vi "SMain.vi"() -> ()   [LabVIEW 2011] (continued)
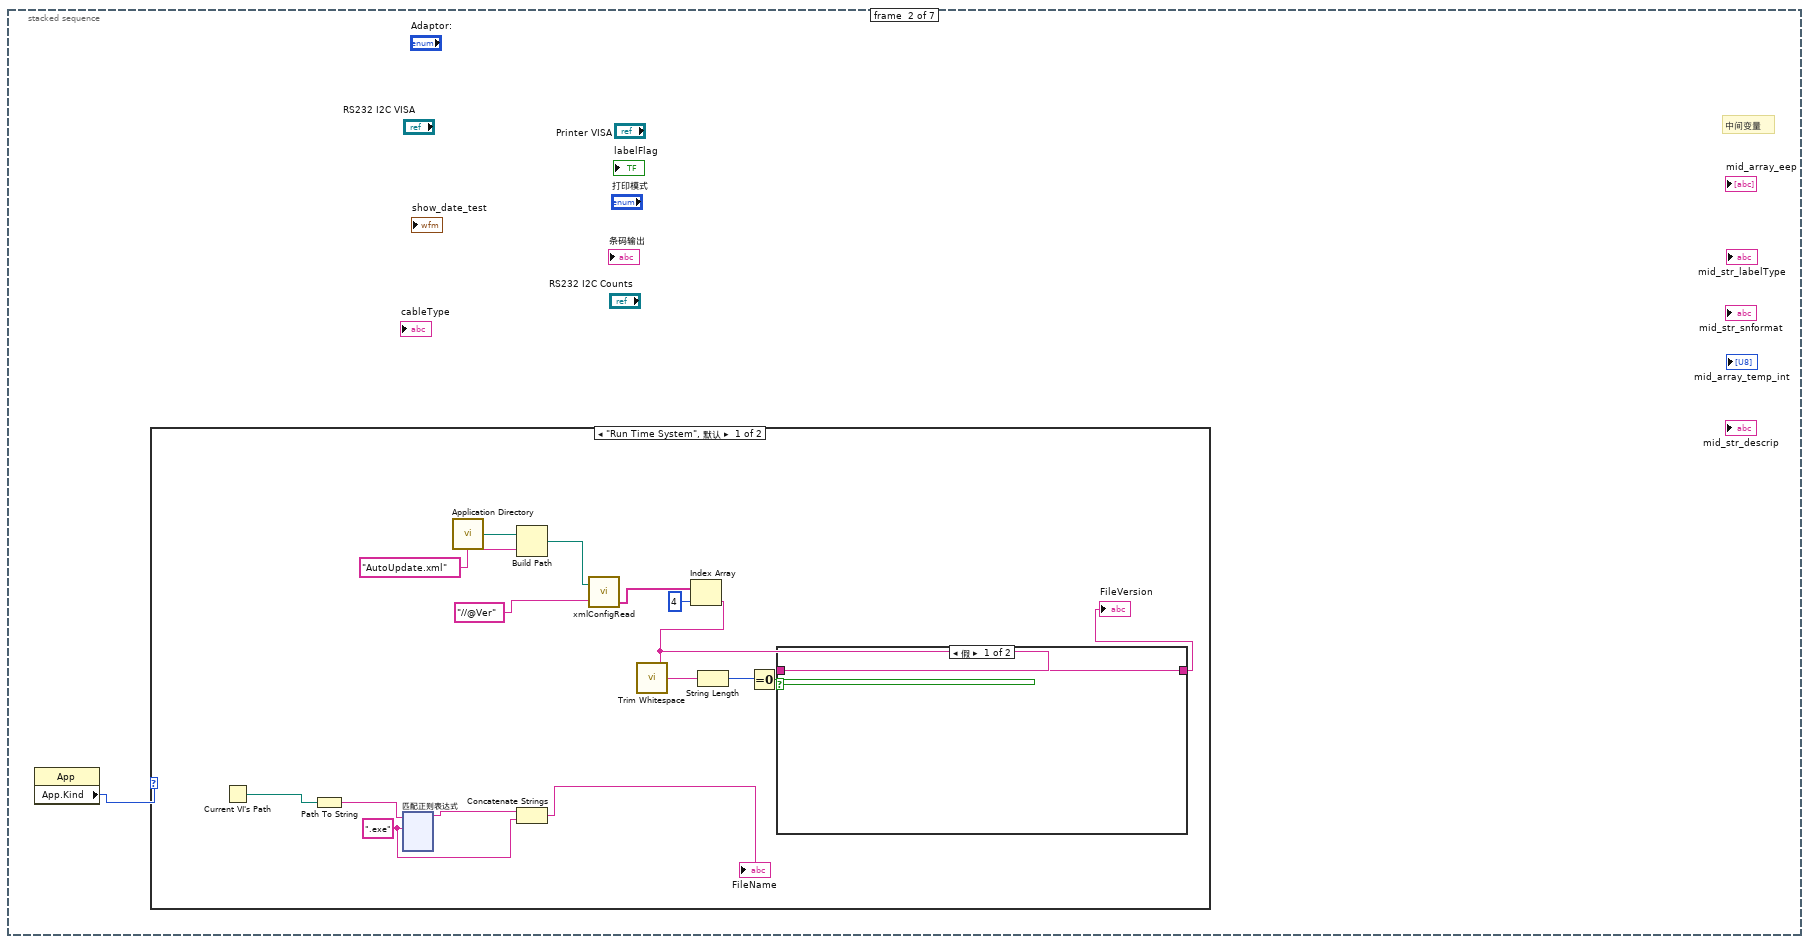
[diagram p4: hidden frame]
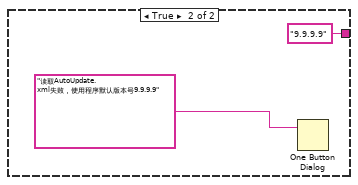
[diagram p5: hidden frame]
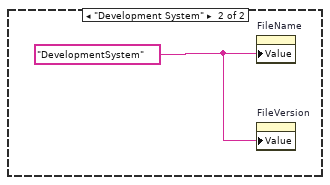
[diagram p6: hidden frame]
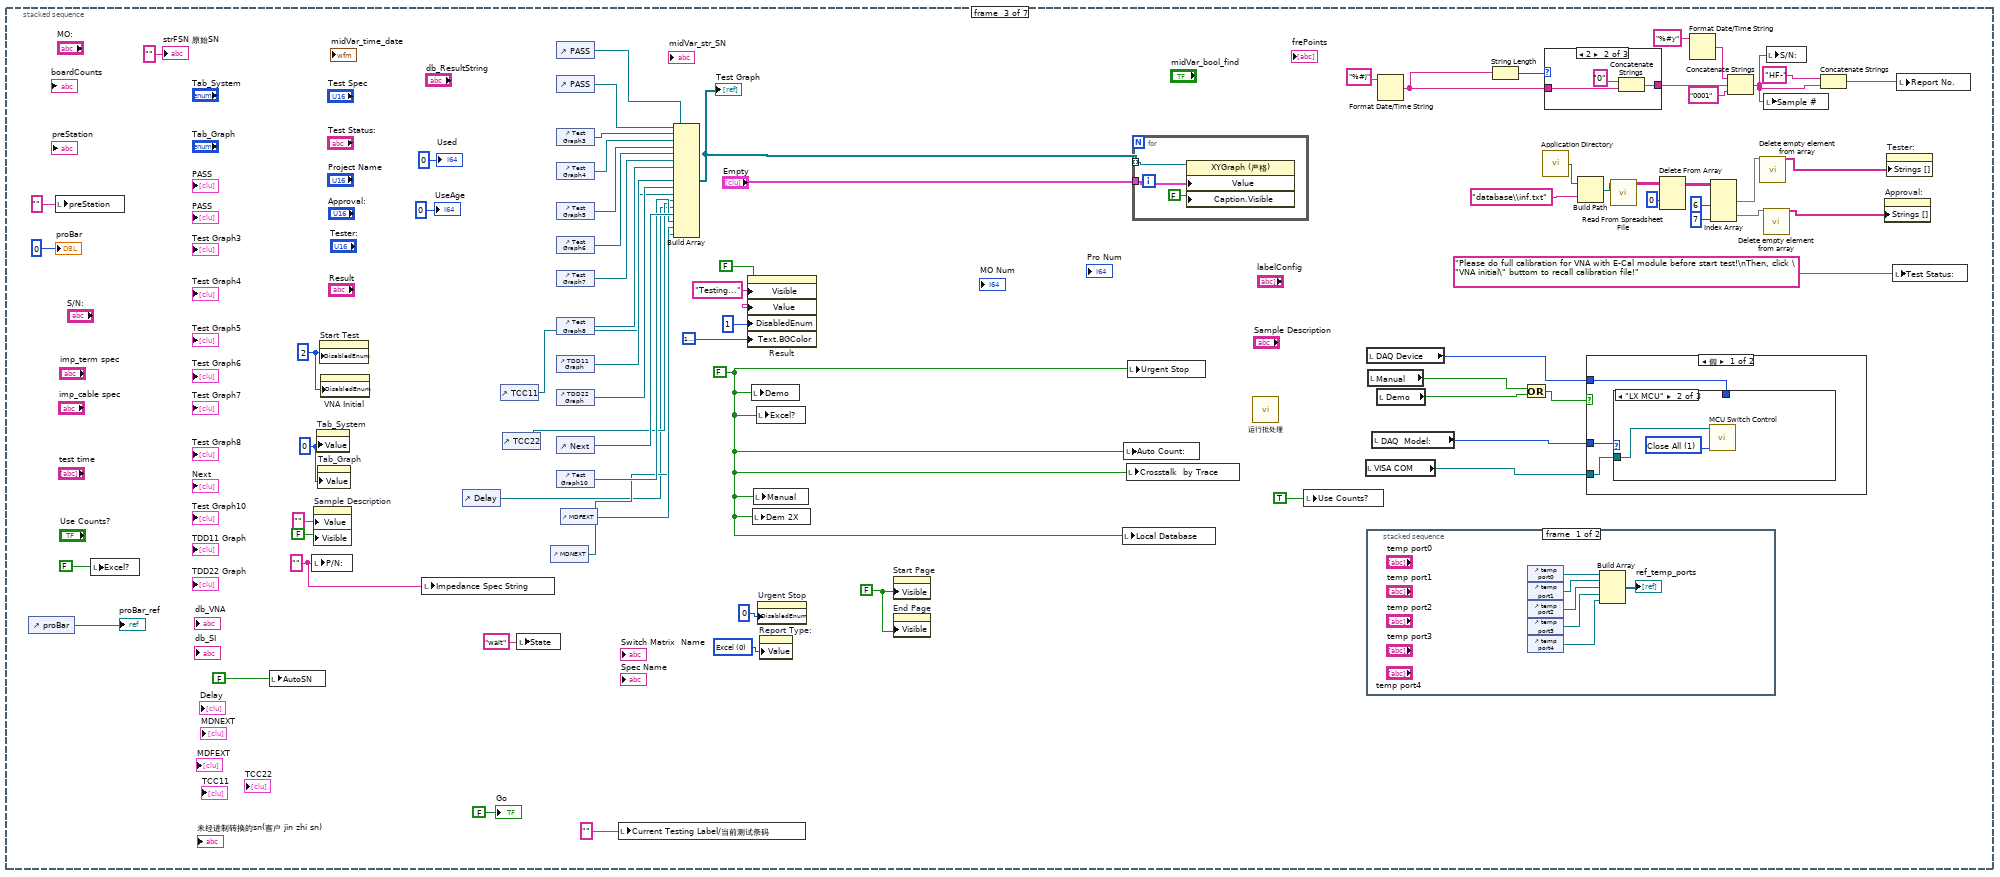
[diagram p7: hidden frame]
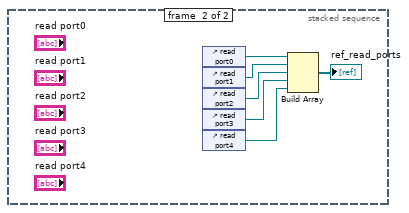
[diagram p8: hidden frame]
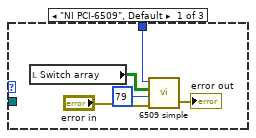
[diagram p9: hidden frame]
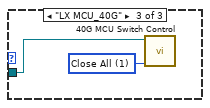
[diagram p10: hidden frame]
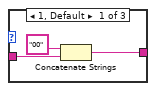
[diagram p12: hidden frame]
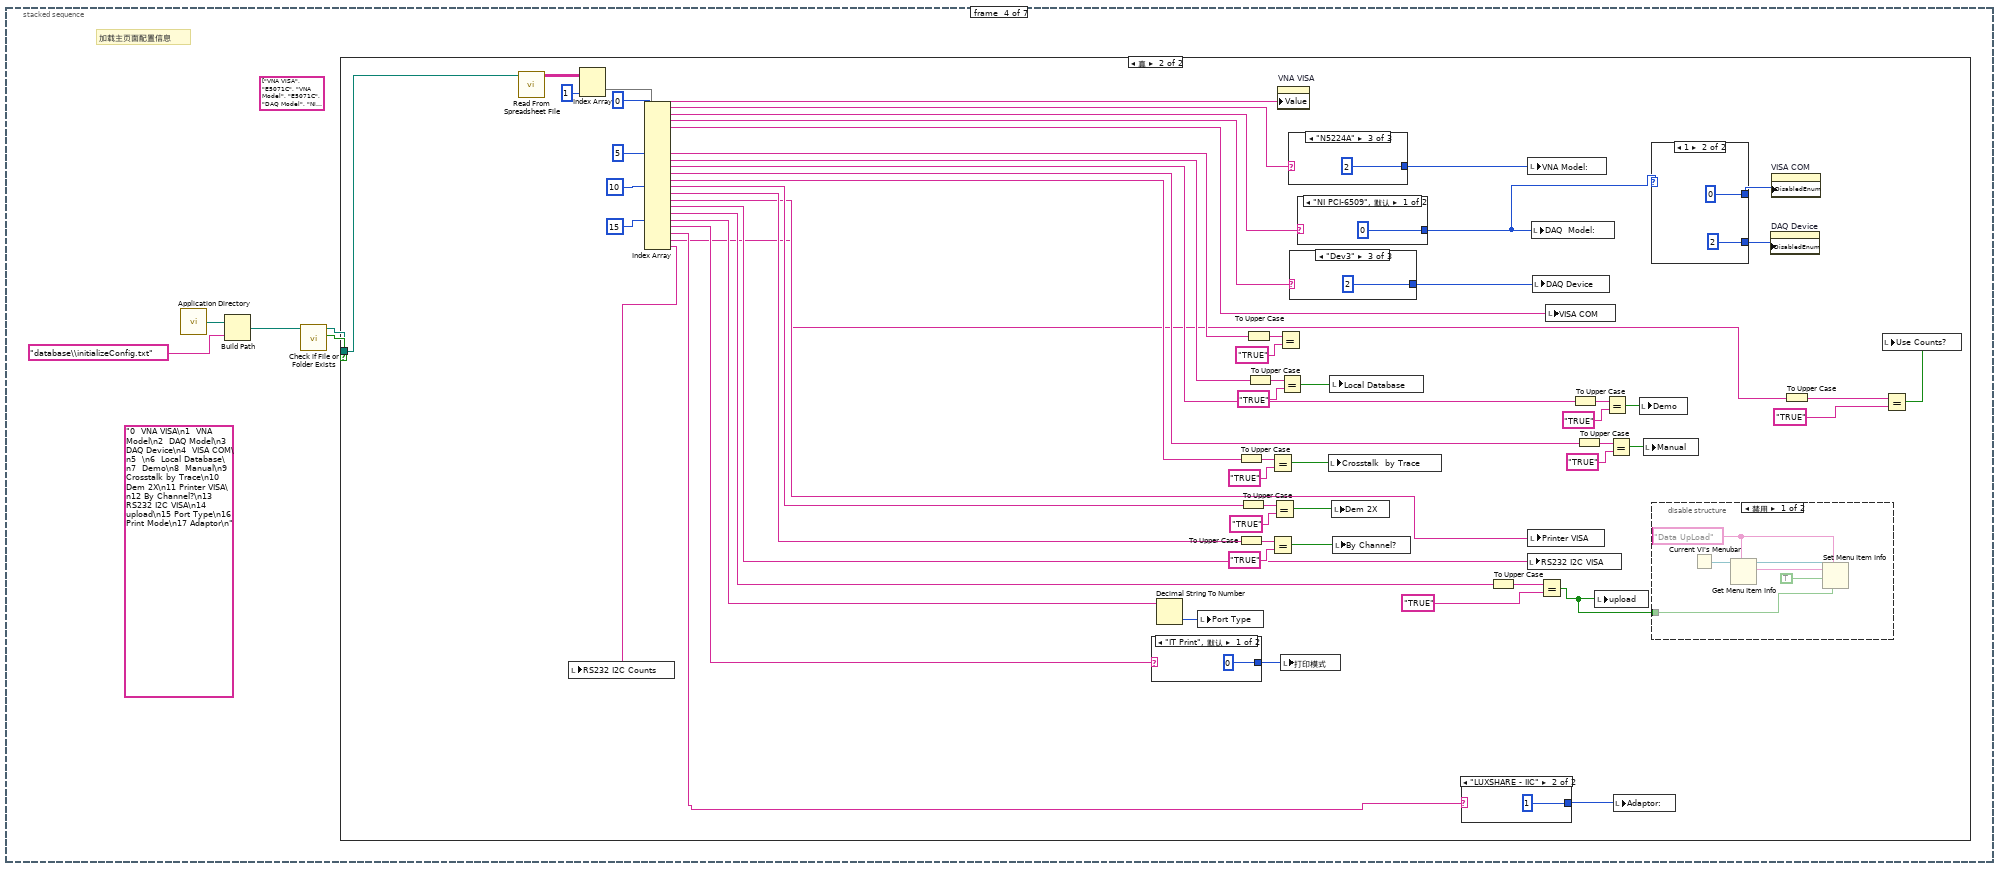
[diagram p14: hidden frame]
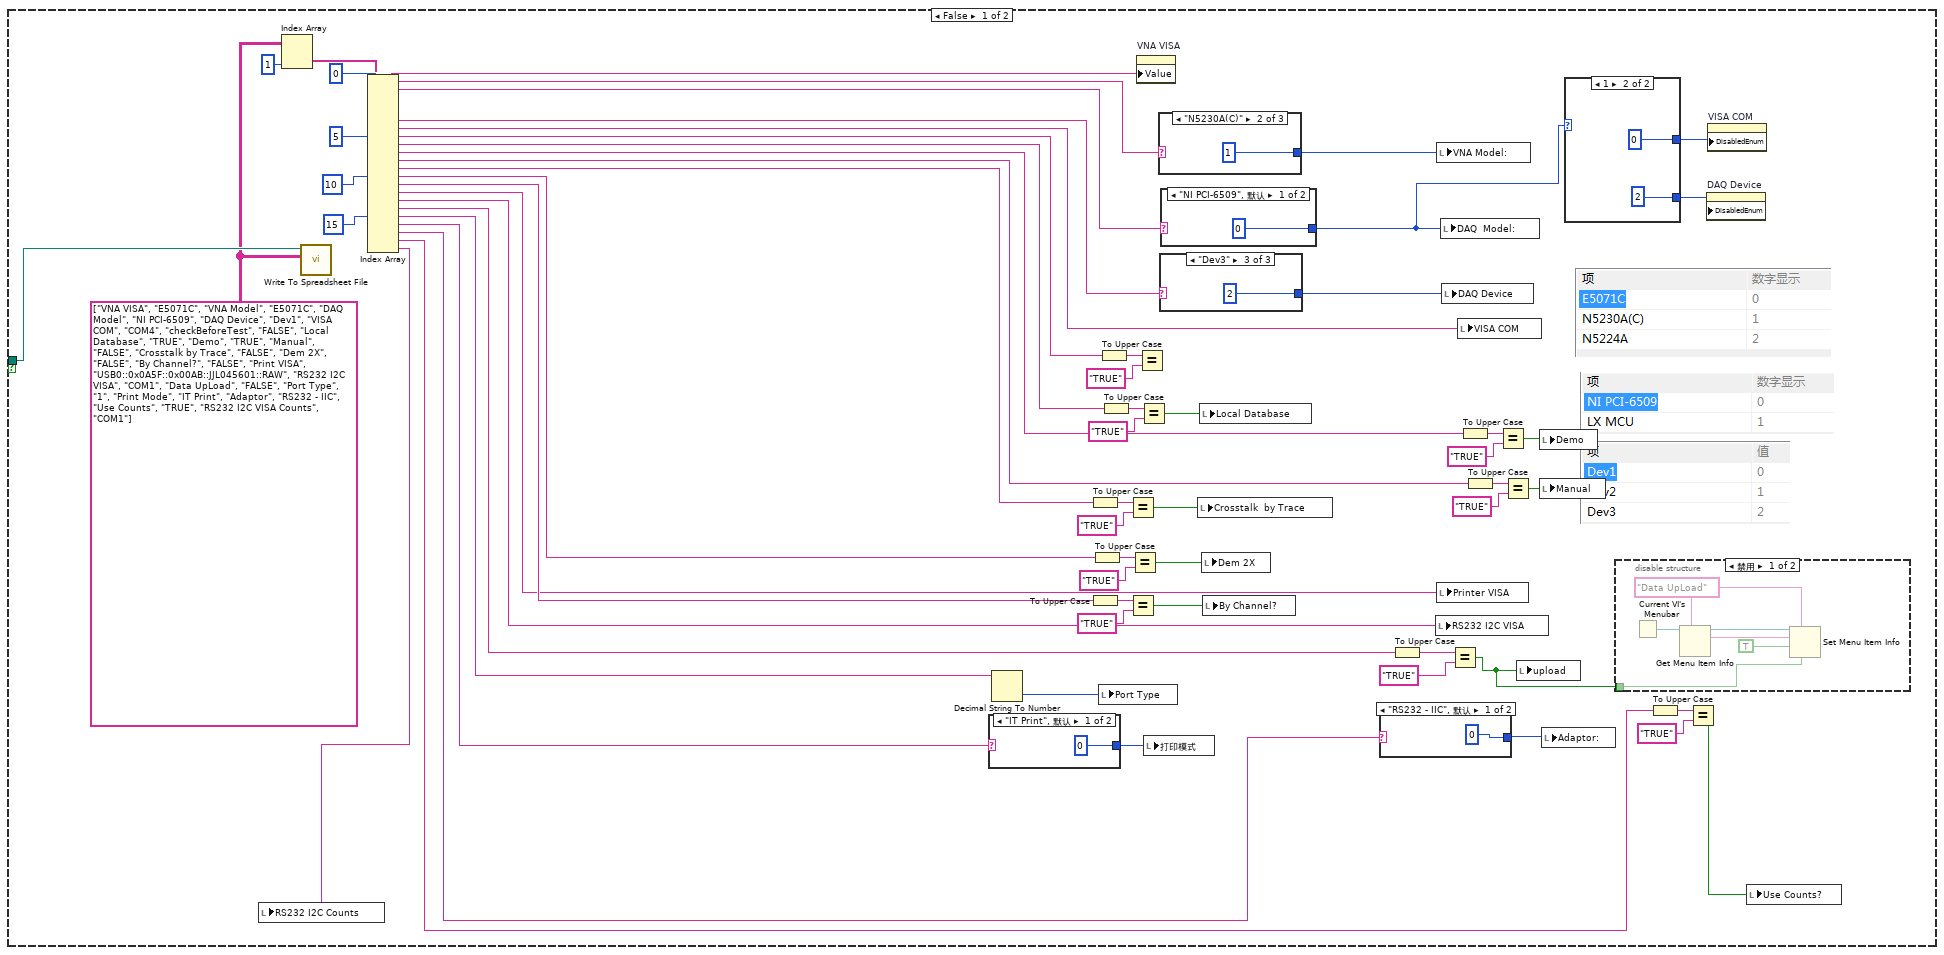
[diagram p15: hidden frame]
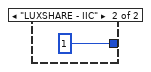
[diagram p17: hidden frame]
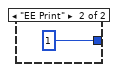
[diagram p18: hidden frame]
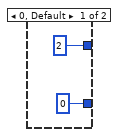
[diagram p19: hidden frame]
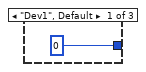
[diagram p20: hidden frame]
                                n1435 = call "getLabelConfigFromSQL.vi"("input_str_labelType"=w2252, "DB"=w2242) -> ("show_array"=w2246:string[])
                                n1436 = local write "mid_array_eep"(w2254) -> ()
                                n1437 = case shown="\"10\"" w2258 {
                                tunnel: w2253 -> [w2261 w2264 _]
                                tunnel: [2 ("索引") 2 ("索引") 0 ("索引")] -> w2247
                                frame "00", "01", Default {
                                n1438 = One Button Dialog(message=w2261) -> ()  [unwired: 1 in, 1 out]
                                n1439 = local write "midVar_bool_find"(FALSE ("midVar_bool_find")) -> ()
                                }
                                frame "10" {
                                n1440 = One Button Dialog(message=w2264) -> ()  [unwired: 1 in, 1 out]
                                n1441 = local write "midVar_bool_find"(FALSE ("midVar_bool_find")) -> ()
                                }
                                frame "11" {
                                n1442 = local write "midVar_bool_find"(TRUE ("midVar_bool_find")) -> ()
                                }
                                }
                                n1443 = Decimal String To Number(string=w2245) -> (number=→"DateCode8Value_0X30":i32)  [unwired: 2 in, 1 out]
                                n1444 = Index Array(array=w2246, index #1=0 ("索引"), index #2=11 ("索引")) -> (element #1=w2248:string, element #2=w2249:string)
                                n1445 = local write "mid_str_snformat"(w2249) -> ()
                                n1446 = local write "labelConfig"(w2246) -> ()
                                n1447 = local write "mid_str_descrip"(w2248) -> ()
                                n1448 = property on="Start Test" class="Bool"("DisabledEnum"=w2247) -> ()  [unwired: 2 in, 2 out]
                                n1449 = property on="VNA Initial" class="Bool"("DisabledEnum"=w2247) -> ()  [unwired: 2 in, 2 out]
                              }
                              frame True {
                                n1450 = Index Array(array=w2269, index #1=13 ("索引"), index #2=14 ("索引")) -> (element #1=w2268:string, element #2=w2271:string)
                                n1451 = local read "P/N:"() -> (w2274:string)
                                n1452 = local write "mid_str_snformat"(w2271) -> ()
                                n1453 = local write "mid_str_labelType"(w2268) -> ()
                                n1454 = call "littleVI_4_readLocalEEPROMFile.vi"("input_PN"=w2274) -> ("show_eeprom"=w2273:string[][])  [unwired: 10 in]
                                n1455 = local write "mid_str_descrip"("" ("mid_str_descrip")) -> ()
                                n1456 = local write "mid_array_eep"(w2273) -> ()
                              }
                            }
                          }
                        }
                        "limitSpec" <- w2235
                      }
                      frame #5 {
                        n1457 = call "Detailed Project Information.vi"("Project  Information Input"=w2302) -> ("TDR Setting2"=→"TDR Setting  2":string[], "minus 2X?"=w2289:bool, "CMP Setting"=w2284:string[], "smooth point"=w2278:i32, "TDR Test Item Name"=→"TDR Test Item Name":string[], "Report Config"=→"Report Config":string[], "ILD Spec No"=→"ILD Spec No":i32, "Report Name"=→"Report Temp. Name":string, "S-para Pair Name"=→"S-para Pair Name":string[], "TDR Setting"=→"TDR Setting":string[], "NEXT Pair Name"=→"NEXT Pair Name":string[], "FEXT Pair Name"=→"FEXT Pair Name":string[], "Diff Test Item Name"=w2287:string[], "Spec Association Col No"=w2293:string[], "Cal File Path"=w2299:string[])  [unwired: 11 in, 1 out]
                        "Spec Association Col No" <- w2293
                        "smooth point" <- w2278
                        "Diff Test Item smooth" <- w2287
                        n1458 = local write "Dem 2X"(w2289) -> ()
                        n1459 = Index Array(array=w2299, index=0 ("索引")) -> (element=→"Cal File Path":string)
                        n1460 = for {
                          tunnel: w2287 -> [w2312] mode=indexing
                          tunnel: [w2309] -> w2281 mode=indexing
                          tunnel: [w2306] -> w2280 mode=indexing
                          n1461 = Search and Replace String(input string=w2312, search string=",smooth" ("搜索字符串"), replace string="" ("替换字符串(\"\")")) -> (result string=w2309:string, number of replacements=w2307:i32)  [unwired: 5 in, 2 out]
                          n1462 = Equal?(x=w2307, y=1) -> (x = y?=w2306:bool)
                        }
                        "Diff Test Item Name" <- w2281
                        n1463 = Decimal String To Number(string=w2293) -> (number=→"Spec _Col":i32[])  [unwired: 2 in, 1 out]
                        n1464 = control-ref of="Tab_Graph"() -> (w2305:refnum<vi>)
                        n1465 = call "Tap Title Modflication.vi"("Test Item Name"=w2287, "Tab_Graph"=w2305) -> ()  [unwired: 10 in]
                        n1466 = call "TestItemCount.vi"("Testitems"=w2287) -> ("Count"=→"Count":i16)
                        n1467 = Index Array(array=w2284, index=0 ("索引")) -> (element=→"CMP setting":string)
                        n1468 = call "Divide Test Items.vi"("Test Item Name"=w2281) -> ("Crosstalk  Item List"=→"Crosstalk Item List":string[], "S-Para Item List"=→"S-Para Item List":string[])  [unwired: 9 in]
                        n1469 = call "getSparaConfig.vi"("Spec Associate"=w2279, "different"=w2281, "smooth"=w2280, "smoothPoints"=w2278) -> ("sPara"=w2277:T3[], "extPara"=w2276:T3[])  [unwired: 10 in]
                        n1470 = Insert Into Array(array=w2277, new element=w2276) -> (→"sSpec":T3[])  [unwired: 1 in]
                      }
                      frame #6 {
                        n1471 = local read "TDR Setting"() -> (w2336:string[])
                        n1472 = Index Array(array=w2336) -> (element #1=w2335:string, element #2=w2334:string, element #3=w2333:string, element #4=w2332:string, element #5=w2330:string, element #6=w2329:string, element #7=w2328:string, element #8=→"Fix Delay(ns)":string, element #9=w2318:string, element #10=w2321:string)  [unwired: 10 in]
                        n1473 = Decimal String To Number(string=w2318) -> (number=→"Skew Spec(ps)":i32)  [unwired: 2 in, 1 out]
                        n1474 = Fract/Exp String To Number(string=w2334) -> (number=w2325:dbl)  [unwired: 3 in, 1 out]
                        n1475 = Fract/Exp String To Number(string=w2335) -> (number=w2326:dbl)  [unwired: 3 in, 1 out]
                        n1476 = Decimal String To Number(string=w2333) -> (number=w2324:i32)  [unwired: 2 in, 1 out]
                        n1477 = Spreadsheet String To Array(format string="%s" ("格式字符串"), spreadsheet string=w2321, array type (2D Dbl)=dbl[] []) -> (array=→"2X IL":dbl[])  [unwired: 1 in]
                        n1478 = Fract/Exp String To Number(string=w2332) -> (number=w2315:dbl)  [unwired: 3 in, 1 out]
                        n1479 = Equal?(x=w2329, y="1") -> (x = y?=w2327:bool)
                        n1480 = Fract/Exp String To Number(string=w2330) -> (number=w2323:dbl)  [unwired: 3 in, 1 out]
                        n1481 = local write "Impedance Spec String"(w2328) -> ()
                        n1482 = local write "Start TimeNs"(w2326) -> ()
                        n1483 = local write "StopTimeNs"(w2325) -> ()
                        n1484 = local write "Data Points"(w2324) -> ()
                        n1485 = local write "Filter Risetime(ps)"(w2315) -> ()
                        n1486 = local write "Compensation(ohm)"(w2323) -> ()
                        n1487 = local write "Impedance Filter"(w2327) -> ()
                        n1488 = Greater?(x=w2315, y=65.0) -> (0:w2313:bool)
                        n1489 = case shown="真" w2313 {
                          frame False {
                          }
                          frame True {
                            n1490 = One Button Dialog(message="risetime时间大于65，请联系钟波\n或方羽确认是否正确！") -> ()  [unwired: 1 in, 1 out]
                          }
                        }
                      }
                      frame #7 {
                        n1491 = local read "TDR Setting  2"() -> (w2359:string[])
                        n1492 = Index Array(array=w2359) -> (element #1=w2358:string, element #2=w2357:string, element #3=w2356:string, element #4=w2355:string, element #5=w2353:string, element #6=w2352:string, element #7=w2351:string, element #8=→"Fix Delay(ns)  2":string, element #9=w2340:string, element #10=w2343:string)  [unwired: 10 in]
                        n1493 = Decimal String To Number(string=w2340) -> (number=→"Skew Spec(ps) 2":i32)  [unwired: 2 in, 1 out]
                        n1494 = Fract/Exp String To Number(string=w2357) -> (number=w2348:dbl)  [unwired: 3 in, 1 out]
                        n1495 = Fract/Exp String To Number(string=w2358) -> (number=w2349:dbl)  [unwired: 3 in, 1 out]
                        n1496 = Decimal String To Number(string=w2356) -> (number=w2347:i32)  [unwired: 2 in, 1 out]
                        n1497 = Spreadsheet String To Array(format string="%s" ("格式字符串"), spreadsheet string=w2343, array type (2D Dbl)=dbl[] []) -> (array=→"2X IL 2":dbl[])  [unwired: 1 in]
                        n1498 = Fract/Exp String To Number(string=w2355) -> (number=w2346:dbl)  [unwired: 3 in, 1 out]
                        n1499 = Equal?(x=w2352, y="1") -> (x = y?=w2350:bool)
                        n1500 = Fract/Exp String To Number(string=w2353) -> (number=w2345:dbl)  [unwired: 3 in, 1 out]
                        n1501 = local write "Impedance Spec String 2"(w2351) -> ()
                        n1502 = local write "Start TimeNs 2"(w2349) -> ()
                        n1503 = local write "StopTimeNs 2"(w2348) -> ()
                        n1504 = local write "Filter Risetime(ps) 2"(w2346) -> ()
                        n1505 = local write "Data Points 2"(w2347) -> ()
                        n1506 = local write "Compensation(ohm) 2"(w2345) -> ()
                        n1507 = local write "Impedance Filter 2"(w2350) -> ()
                      }
                      frame #8 {
                        n1508 = call "(0,1)to(true,false) by data.vi"("Switch data"=w2361) -> ("Switch array"=→"Switch array":bool[][])  [unwired: 2 in]
                      }
                      frame #9 {
                        w2364 = 8 ("y")
                        n1509 = disable-structure shown="禁用" {
                          frame Disabled {
                            n1510 = local read "Diff Test Item Name"() -> (w2369:string[])
                            n1511 = call "Divide Test Items.vi"("Test Item Name"=w2369) -> ()  [unwired: 9 in, 2 out]
                          }
                          frame Enabled {
                          }
                        }
                        n1512 = local read "S-Para Item List"() -> (w2362:string[])
                        n1513 = Array Size(array=w2362) -> (size(s)=w2366:i32)
                        n1514 = local read "Test Graph"() -> (w2368:refnum<vi>[])
                        n1515 = local read "Empty"() -> (w2367:cluster{"Horz Time array":dbl[], "Y":dbl[]}[])
                        n1516 = Less Or Equal?(x=w2366, y=w2364) -> (x <= y?=w2365:bool)
                        n1517 = Select(t=w2366, s=w2365, f=w2364) -> (s? t:f=w2363:i32)
                        n1518 = for {
                          tunnel: w2368 -> [w2375] mode=indexing
                          tunnel: w2367 -> [w2374]
                          tunnel: w2363 -> [w2371]
                          tunnel: w2362 -> [w2373]
                          i -> [w2370]
                          n1519 = Index Array(array=w2373, index=w2370) -> (element=w2372:string)
                          n1520 = Less?(x=w2370, y=w2371) -> (x < y?=w2376:bool)
                          n1521 = case shown="假" w2376 {
                            tunnel: w2375 -> [w2378 w2382]
                            tunnel: w2374 -> [w2377 w2381]
                            tunnel: w2372 -> [_ w2380]
                            frame False {
                              n1522 = property class="XYGraph (严格)"(reference=w2378, "Value"=w2377, "Caption.Visible"=FALSE ("标题.可见")) -> ()  [unwired: 1 in, 2 out]
                            }
                            frame True {
                              n1523 = property class="XYGraph (严格)"(reference=w2382, "Value"=w2381, "Caption.Visible"=TRUE ("标题.可见"), "Caption.Text"=w2380) -> ()  [unwired: 1 in, 2 out]
                            }
                          }
                        }
                      }
                      frame #10 {
                        n1524 = case shown="假" w2384 {
                          frame False {
                            n1525 = stacked-sequence {
                              seq-local: [_ w2386 _] -> [_ _ w2393]
                              frame #0 {
                                n1526 = local write "Test Status:"("Initializing VNA ....." ("Test Status:")) -> ()
                              }
                              frame #1 {
                                n1527 = local read "Cal File Path"() -> (w2387:string)
                                n1528 = local read "VNA Model:"() -> (w2388:enum16{"E5071C", "N5230A(C)", "N5224A"})
                                n1529 = local read "VNA VISA"() -> (w2389:refnum<visa-resource-name>)
                                n1530 = call "VNA Initial.vi"("Cal File Name Path"=w2387, "VNA Model:"=w2388, "VNA VISA"=w2389) -> ("Connect?"=w2386:bool)  [unwired: 8 in]
                              }
                              frame #2 {
                                n1531 = Select(t=0 ("索引"), s=w2393, f=2 ("索引")) -> (s? t:f=w2394:i32)
                                n1532 = property on="Start Test" class="Bool"("DisabledEnum"=w2394) -> ()  [unwired: 2 in, 2 out]
                                n1533 = property on="VNA Initial" class="Bool"("DisabledEnum"=w2394) -> ()  [unwired: 2 in, 2 out]
                                n1534 = Select(t="VNA Initialization Finished!\nPlease Slect Correct Project & Test Spec & Switch Matrix to Start Testing " ("Test Status:"), s=w2393, f="VNA Initialization Not Be Finished!\nPlease Check VNA Connection!" ("Test Status:")) -> (s? t:f=w2391:string)
                                n1535 = local write "Test Status:"(w2391) -> ()
                              }
                            }
                          }
                          frame True {
                            n1536 = property on="Start Test" class="Bool"("DisabledEnum"=0 ("索引")) -> ()  [unwired: 2 in, 2 out]
                            n1537 = local write "Test Status:"("Please do full calibration for VNA with E-Cal module before start test!\nThen, click \"VNA initial\" buttom to recall calibration file!" ("Test Status:")) -> ()
                          }
                        }
                      }
                      frame #11 {
                        (unwired) "Initializing VNA ....." ("Test Status:")
                        # "增加华为完整XML生成料号配置文件读取功能"
                        n1538 = call <vilib>:"Application Directory.vi"() -> ("Application Directory"=w2404:path)
                        n1539 = Build Path(base path=w2404, name or relative path="Database\\FigoConfig.xml") -> (appended path=w2402:path)
                        n1540 = call <vilib>:"Check if File or Folder Exists.vi"("path"=w2402) -> ("file or folder exists?"=w2401:bool, "dup path"=w2400:path)  [unwired: 8 in, 1 out]
                        n1541 = case shown="真" w2401 {
                          tunnel: w2400 -> [w2408 w2423]
                          tunnel: w2399 -> [_ w2428]
                          frame False {
                            n1542 = Path To String(path=w2408) -> (string=w2407:string)
                            n1543 = Concatenate Strings("文件" ("字符串"), w2407, "加载失败，将使用默认值" ("字符串")) -> (w2405:string)
                            n1544 = One Button Dialog(message=w2405) -> ()  [unwired: 1 in, 1 out]
                          }
                          frame True {
                            n1545 = local read "打印模式"() -> (w2426:enum16{"IT Print", "EE Print"})
                            n1546 = call "校验信息获取.vi"("料号"=w2428, "path to XML document"=w2423) -> ("校验信息"=→"校验信息":T7)  [unwired: 9 in]
                            n1547 = call "xmlConfigRead.vi"("path to XML document"=w2423, "XPath expression"="//PartNoWithFullXml/PartNo/@Name") -> ("OutParaArray"=w2427:string[])  [unwired: 2 out]
                            n1548 = local read "P/N:"() -> (w2425:string)
                            n1549 = call "xmlConfigRead.vi"("path to XML document"=w2423, "XPath expression"="//PartNoWith2X/PartNo/@Name") -> ("OutParaArray"=w2433:string[])  [unwired: 2 out]
                            n1550 = call "EEUpload.vi"("PN"=w2425, "打印模式"=w2426, "xmlConfigPath"=w2423) -> ("EEUPLOAD"=→"EEUPLOAD":bool)  [unwired: 6 in, 2 out]
                            n1551 = Search 1D Array(1D array=w2427, element=w2425) -> (index of element=w2439:i32)  [unwired: 1 in]
                            n1552 = Search 1D Array(1D array=w2433, element=w2425) -> (index of element=w2432:i32)  [unwired: 1 in]
                            n1553 = Equal?(x=w2439, y=-1) -> (x = y?=w2437:bool)
                            n1554 = Not Equal?(x=w2432, y=-1) -> (x != y?=w2430:bool)
                            "2x equalize" <- w2430
                            n1555 = case shown="假" w2430 {
                              frame False {
                                n1556 = local write "Test Status:"("ILD_15将会采用与SDD21设定方式进行计算") -> ()
                              }
                              frame True {
                                n1557 = local write "Test Status:"("ILD_15将会加上2X夹具值后进行计算") -> ()
                              }
                            }
                            n1558 = Not(x=w2437) -> (.not. x?=w2436:bool)
                            "FullXml" <- w2436
                            n1559 = case shown="真" w2436 {
                              tunnel: w2423 -> [_ w2462]
                              tunnel: w2425 -> [_ w2463]
                              frame False {
                                n1560 = local read "Test Status:"() -> (w2445:string)
                                n1561 = Concatenate Strings(w2445, "\n", "将生成精简的XML文件") -> (w2442:string)
                                n1562 = local write "Test Status:"(w2442) -> ()
                              }
                              frame True {
                                n1563 = Search and Replace String(input string="//PartNoWithFullXml/PartNo[@Name='@Name@']/@*" ("XPath expression"), search string="@Name@" ("搜索字符串"), replace string=w2463) -> (result string=w2467:string)  [unwired: 5 in, 3 out]
                                n1564 = call "xmlConfigRead.vi"("path to XML document"=w2462, "XPath expression"=w2467) -> ("OutParaArray"=w2466:string[])  [unwired: 2 out]
                                n1565 = Index Array(array=w2466, index #1=1 ("索引"), index #2=2 ("索引"), index #3=3 ("索引"), index #4=4 ("索引")) -> (element #1=w2458:string, element #2=→"PN TYpe":string, element #3=w2448:string, element #4=w2447:string)
                                n1566 = local read "Test Status:"() -> (w2453:string)
                                n1567 = To Upper Case(1:w2458) -> (0:w2459:string)
                                n1568 = Decimal String To Number(string=w2448) -> (number=→"width1":i32)  [unwired: 2 in, 1 out]
                                n1569 = Decimal String To Number(string=w2447) -> (number=→"width2":i32)  [unwired: 2 in, 1 out]
                                n1570 = Equal?(x=w2459, y="TRUE") -> (x = y?=→"auto get refer point":bool)
                                n1571 = Concatenate Strings(w2453, "\n", "将生成完整频点的XML文件的华为料号，是否生成依赖FullXML?的设定") -> (w2450:string)
                                n1572 = local write "Test Status:"(w2450) -> ()
                              }
                            }
                            n1573 = call "xmlConfigRead.vi"("path to XML document"=w2423, "XPath expression"="//UploadPara/*") -> ("OutParaArray"=w2421:string[])  [unwired: 2 out]
                            n1574 = Index Array(array=w2421) -> (element #1=w2419:string, element #2=w2418:string, element #3=w2417:string, element #4=w2416:string, element #5=w2415:string, element #6=w2414:string, element #7=w2413:string, element #8=w2411:string, element #9=w2410:string)  [unwired: 9 in]
                            n1575 = Bundle By Name(cluster=T1 {"NetCmdHW"="", "NetPathHW"="", "NetCmdCompress"="", "NetPathCompress1"="", "NetPathCompress2"="", "AlarmDisplay"="", "Synchronous"="", "NetTemppath"="", "NetLocalpath"=""} ("UploadPara"), "NetCmdHW"=w2419, "NetPathHW"=w2418, "NetCmdCompress"=w2417, "NetPathCompress1"=w2416, "NetPathCompress2"=w2415, "AlarmDisplay"=w2414, "Synchronous"=w2413, "NetTemppath"=w2411, "NetLocalpath"=w2410) -> (→"uploadPara":T1)
                            n1576 = call "createFolder.vi"("字符串"=w2411) -> ()  [unwired: 11 in]
                            n1577 = call "createFolder.vi"("字符串"=w2410) -> ()  [unwired: 11 in]
                          }
                        }
                      }
                      frame #12 {
                        n1578 = Index Array(array=w2475, index=2 ("索引")) -> (element=w2473:string)
                        n1579 = To Upper Case(1:w2473) -> (0:w2472:string)
                        n1580 = Equal?(x=w2472, y="HUAWEI") -> (x = y?=w2470:bool)
                        "PassCount?" <- w2470
                        n1581 = property on="Passed" class="DigNum (严格)"("Visible"=w2470) -> ()  [unwired: 2 in, 2 out]
                        n1582 = property on="Total" class="DigNum (严格)"("Visible"=w2470) -> ()  [unwired: 2 in, 2 out]
                        n1583 = property on="Failed" class="DigNum (严格)"("Visible"=w2470) -> ()  [unwired: 2 in, 2 out]
                        n1584 = property on="ratio" class="DigNum (严格)"("Visible"=w2470) -> ()  [unwired: 2 in, 2 out]
                        n1585 = case shown="真" w2470 {
                          tunnel: w2469 -> [_ w2487]
                          frame False {
                          }
                          frame True {
                            n1586 = Format Date/Time String(time format string (%c)="%Y%m%d" ("时间格式字符串(%c)")) -> (date/time string=w2484:string)  [unwired: 2 in]
                            n1587 = call <vilib>:"Application Directory.vi"() -> ("Application Directory"=w2490:path)
                            n1588 = Concatenate Strings("DataBase\\" ("字符串"), w2487, "\\" ("字符串"), w2484, ".xml" ("字符串")) -> (w2482:string)
                            n1589 = Build Path(base path=w2490, name or relative path=w2482) -> (appended path=w2489:path)
                            "CountXmlPath" <- w2489
                            n1590 = call <vilib>:"Check if File or Folder Exists.vi"("path"=w2489) -> ("file or folder exists?"=w2481:bool, "dup path"=w2480:path)  [unwired: 8 in, 1 out]
                            n1591 = case shown="真" w2481 {
                              tunnel: w2480 -> [w2491 w2510]
                              tunnel: [0 w2506] -> w2479
                              tunnel: [0 w2504] -> w2478
                              tunnel: [0 w2503] -> w2477
                              tunnel: [0.0 w2502] -> w2476
                              frame False {
                                n1592 = stacked-sequence {
                                tunnel: w2491 -> [w2499 w2501]
                                frame #0 {
                                n1593 = Strip Path(path=w2499) -> (stripped path=w2498:path)  [unwired: 1 out]
                                n1594 = call <vilib>:"Check if File or Folder Exists.vi"("path"=w2498) -> ("file or folder exists?"=w2497:bool, "dup path"=w2496:path)  [unwired: 8 in, 1 out]
                                n1595 = case shown="假" w2497 {
                                tunnel: w2496 -> [w2500 _]
                                frame False {
                                n1596 = Create Folder(path (use dialog)=w2500) -> ()  [unwired: 2 in, 3 out]
                                }
                                frame True {
                                }
                                }
                                }
                                frame #1 {
                                n1597 = call "xmlNodecreate.vi"("path"=w2501) -> ()  [unwired: 3 in, 1 out]
                                }
                                }
                              }
                              frame True {
                                # "增加华为完整XML生成料号配置文件读取功能"
                                n1598 = call "xmlConfigRead.vi"("path to XML document"=w2510, "XPath expression"="//FailedSN/*") -> ("OutParaArray"=w2507:string[])  [unwired: 2 out]
                                n1599 = call "xmlConfigRead.vi"("path to XML document"=w2510, "XPath expression"="//PassedSN/*") -> ("OutParaArray"=w2508:string[])  [unwired: 2 out]
                                n1600 = Array Size(array=w2508) -> (size(s)=w2506:i32)
                                n1601 = Array Size(array=w2507) -> (size(s)=w2504:i32)
                                n1602 = Add(x=w2504, y=w2506) -> (x+y=w2503:i32)
                                n1603 = Equal To 0?(x=w2503) -> (x = 0?=w2505:bool)
                                n1604 = case shown="假" w2505 {
                                tunnel: w2504 -> [w2516 _]
                                tunnel: w2503 -> [w2515 _]
                                tunnel: [w2512 0.0] -> w2502
                                frame False {
                                n1605 = Divide(x=w2516, y=w2515) -> (x/y=w2514:dbl)
                                n1606 = Multiply(x=w2514, y=100.0) -> (x*y=w2512:dbl)
                                }
                                frame True {
                                }
                                }
                              }
                            }
                            "Total" <- w2477
                            "Passed" <- w2479
                            "Failed" <- w2478
                            "ratio" <- w2476
                          }
                        }
                      }
                      frame #13 {
                        n1607 = call "getDebugMode.vi"() -> ("debugMode"=w2518:bool)  [unwired: 11 in]
                        n1608 = case shown="真" w2518 {
                          frame False {
                          }
                          frame True {
                            n1609 = One Button Dialog(message="当前模式为debug模式，仅可用于调试用\n请注意" ("消息")) -> ()  [unwired: 1 in, 1 out]
                          }
                        }
                        n1610 = local read "SystemMode"() -> (w2522:string)
                        n1611 = local read "DB1"() -> (w2521:T8)
                        n1612 = call "checkCalistatus.vi"("DBSet"=w2521, "SystemMode"=w2522) -> ("calibrated?"=w2520:bool)  [unwired: 9 in]
                        n1613 = Or(x=w2520, y=w2518) -> (x .or. y?=w2519:bool)
                        n1614 = case shown="真" w2519 {
                          frame False {
                            n1615 = local read "caliDataSelect"() -> (w2524:bool)
                            n1616 = case shown="真" w2524 {
                              frame False {
                                n1617 = One Button Dialog(message="请先选择sampleNo" ("消息")) -> ()  [unwired: 1 in, 1 out]
                                n1618 = property on="Start Test" class="Bool"("DisabledEnum"=T17."Disabled and Grayed Out" ("禁用")) -> ()  [unwired: 2 in, 2 out]
                              }
                              frame True {
                                n1619 = property on="Start Test" class="Bool"("BoolText.Text"="Calibrate" ("布尔文本.文本")) -> ()  [unwired: 2 in, 2 out]
                                n1620 = property on="Start Test" class="Bool"("DisabledEnum"=T17."Enabled" ("禁用")) -> ()  [unwired: 2 in, 2 out]
                                n1621 = One Button Dialog(message="该测试机台当日未校验，测试前需要校验" ("消息")) -> ()  [unwired: 1 in, 1 out]
                                "caliFlag" <- "cali"
                              }
                            }
                          }
                          frame True {
                            n1622 = property on="Start Test" class="Bool"("BoolText.Text"="START TEST" ("布尔文本.文本")) -> ()  [unwired: 2 in, 2 out]
                            n1623 = One Button Dialog(message="该机台已经通过校验，可以开始测试") -> ()  [unwired: 1 in, 1 out]
                            n1624 = local write "caliFlag"("" ("caliFlag")) -> ()
                          }
                        }
                      }
                      frame #14 {
                      }
                    }
                  }
                }
              }
              event "P/N:": Key Down? {
                n1625 = event-data() -> ("Char"=w2535:i16)  [unwired: 1 in, 8 out]
                n1626 = call "aToAchar.vi"("old char"=w2535) -> ("new char"=w2534:dbl)
                n1627 = event-data("Char"=w2534) -> ()  [unwired: 6 in, 1 out]
              }
              event "MO:": Key Down? {
                n1628 = event-data() -> ("Char"=w2536:i16)  [unwired: 1 in, 8 out]
                n1629 = call "aToAchar.vi"("old char"=w2536) -> ("new char"=w2537:dbl)
                n1630 = event-data("Char"=w2537) -> ()  [unwired: 6 in, 1 out]
              }
              event "VNA Initial": Value Change {
                n1631 = event-data() -> ()  [unwired: 1 in, 5 out]
              }
              event Panel Close? {
                n1632 = event-data() -> ()  [unwired: 1 in, 3 out]
                n1633 = call <vilib>:"Application Directory.vi"() -> ("Application Directory"=w2541:path)
                n1634 = Build Path(base path=w2541, name or relative path="Database" ("名称或相对路径")) -> (appended path=w2544:path)
                n1635 = Build Path(base path=w2544, name or relative path="FigoConfig.xml" ("名称或相对路径")) -> (appended path=w2540:path)
                n1636 = call <vilib>:"Check if File or Folder Exists.vi"("path"=w2540) -> ("file or folder exists?"=w2538:bool, "dup path"=w2539:path)  [unwired: 8 in, 1 out]
                n1637 = case shown="真" w2538 {
                  tunnel: w2539 -> [_ w2550]
                  frame False {
                  }
                  frame True {
                    n1638 = local read "P/N:"() -> (w2566:string)
                    n1639 = local read "MO:"() -> (w2567:string)
                    n1640 = Path To String(path=w2550) -> (string=w2553:string)
                    n1641 = call-poly <vilib>:"Load.vi"("path to XML document"=w2550) -> ("DOM document out"=w2562:refnum<k20>, "error out"=w2560:errorcluster)  [unwired: 12 in, 1 out]
                    n1642 = Build Array(w2566, w2567) -> (w2565:string[])
                    n1643 = call <vilib>:"Get All Matched Nodes.vi"("error in (no error)"=w2560, "XPath expression"="//LastPartNo/*", "node in"=w2562) -> ("error out"=w2559:errorcluster, "node result array"=w2564:refnum<k20>[], "node out"=w2561:refnum<k20>)  [unwired: 6 in]
                    n1644 = for {
                      tunnel: w2564 -> [w2572] mode=indexing
                      tunnel: w2565 -> [w2569] mode=indexing
                      shift-right: [w2570] -> w2558
                      shift-left: w2559 -> [w2571]
                      n1645 = call <vilib>:"Set Node Text Content.vi"("error in (no error)"=w2571, "newValue"=w2569, "node in"=w2572) -> ("error out"=w2570:errorcluster)  [unwired: 6 in, 2 out]
                    }
                    n1646 = call <vilib>:"Save.vi"("error in (no error)"=w2558, "XML file path"=w2550, "DOM document in"=w2561) -> ("error out"=w2547:errorcluster)  [unwired: 6 in, 2 out]
                    n1647 = Search and Replace String(replace all?=TRUE ("替换全部？(F)"), input string=w2553, search string="\\" ("搜索字符串"), replace string="\\\\" ("替换字符串(\"\")"), error in=w2547) -> (result string=w2548:string, error out=w2546:errorcluster)  [unwired: 3 in, 2 out]
                    n1648 = constructor class="Operate"(error in=w2546) -> (reference out=w2555:refnum<k24>, error out=w2554:errorcluster)  [unwired: 2 in, 1 out]
                    n1649 = invoke class="Operate" method="xmlFormat"(reference=w2555, error in=w2554, "strFilePath"=w2548) -> (error out=w2545:errorcluster)  [unwired: 1 in, 3 out]
                    n1650 = Unbundle By Name(w2545) -> ("status"=w2557:bool, "source"=w2556:string)  [unwired: 1 out]
                    n1651 = case shown="真" w2557 {
                      tunnel: w2556 -> [_ w2568]
                      frame False {
                      }
                      frame True {
                        n1652 = One Button Dialog(message=w2568) -> ()  [unwired: 1 in, 1 out]
                      }
                    }
                  }
                }
                n1653 = event-data() -> ()  [unwired: 2 in, 1 out]
              }
            }
          }
        }
      }
      n1654 = while {
        stop <- w598 stop-if-true
        n1655 = local read "Urgent Stop"() -> (w598:bool)
        n1656 = Wait (ms)(milliseconds to wait=u32 50 ("等待时间（毫秒）")) -> ()  [unwired: 1 out]
        n1657 = global write "全局.vi" "manual stop"(w598) -> ()
      }
    }
  }
  n1658 = disable-structure shown="禁用" {
    frame Disabled {
    }
    frame Enabled {
    }
  }
